vi "PlayViolins.vi"(11 "Paths to FRFs":path[](array[path])=[path "/Users/crogers/Rogers Dropbox/Chris Rogers/Violin Stuff/Violin Instruments/ME45/ME45 01/TRF/ME45 01 H_001.trf", path "/Users/crogers/Rogers Dropbox/Chris Rogers/Violin Stuff/Violin Instruments/ME45/ME45 02/TRF/ME45 02 H_001.trf", path "/Users/crogers/Rogers Dropbox/Chris Rogers/Violin Stuff/Violin Instruments/ME45/ME45 03/TRF/ME45 03 H_001.trf"]) -> ()   [LabVIEW 2024]
uses:
  <vilib>/Analysis/2dsp.llb/Inverse Complex FFT.vi
  <vilib>/Analysis/2dsp.llb/1D Convolution (DBL).vi
  <vilib>/Analysis/NI_AALPro.lvlib
  <vilib>/Analysis/NI_AALBase.lvlib
panel:
  out "Convolutions 2":waveform(dbl)[](graph)=[{"t0"=timestamp(0 s since 1904-01-01), "dt"=2.0833333333333333e-05, "Y"=array[312010 elements]}, {"t0"=timestamp(0 s since 1904-01-01), "dt"=2.0833333333333333e-05, "Y"=array[312010 elements]}, {"t0"=timestamp(0 s since 1904-01-01), "dt"=2.0833333333333333e-05, "Y"=array[312010 elements]}]
  in  "index 2":i32=48000
  in  "index":i32
  in  "Stop Button":bool
  in  "Play convolution":bool
  out "FRFs":cluster{"t0":dbl, "dt":dbl, "Y":dbl[]}[](graph)=[{"t0"=0.0, "dt"=1.0, "Y"=array[24001 elements]}, {"t0"=0.0, "dt"=1.0, "Y"=array[24001 elements]}, {"t0"=0.0, "dt"=1.0, "Y"=array[24001 elements]}]
  out "Real":T1(graph)
  out "Imaginary":T1(graph)
  in  "Play signal":bool
  in  "Path to signal":path=path "/Users/crogers/Desktop/Joseph_Convolution/1 Tchaikovsky short.wav"
  in  "musical piece":waveform(dbl)[](graph)=[{"t0"=timestamp(0 s since 1904-01-01), "dt"=2.0833333333333333e-05, "Y"=array[288010 elements]}, {"t0"=timestamp(0 s since 1904-01-01), "dt"=2.0833333333333333e-05, "Y"=array[288010 elements]}]
  out "Convolutions":waveform(dbl)[](graph)=[{"t0"=timestamp(0 s since 1904-01-01), "dt"=2.0833333333333333e-05, "Y"=array[312010 elements]}, {"t0"=timestamp(0 s since 1904-01-01), "dt"=2.0833333333333333e-05, "Y"=array[312010 elements]}, {"t0"=timestamp(0 s since 1904-01-01), "dt"=2.0833333333333333e-05, "Y"=array[312010 elements]}]
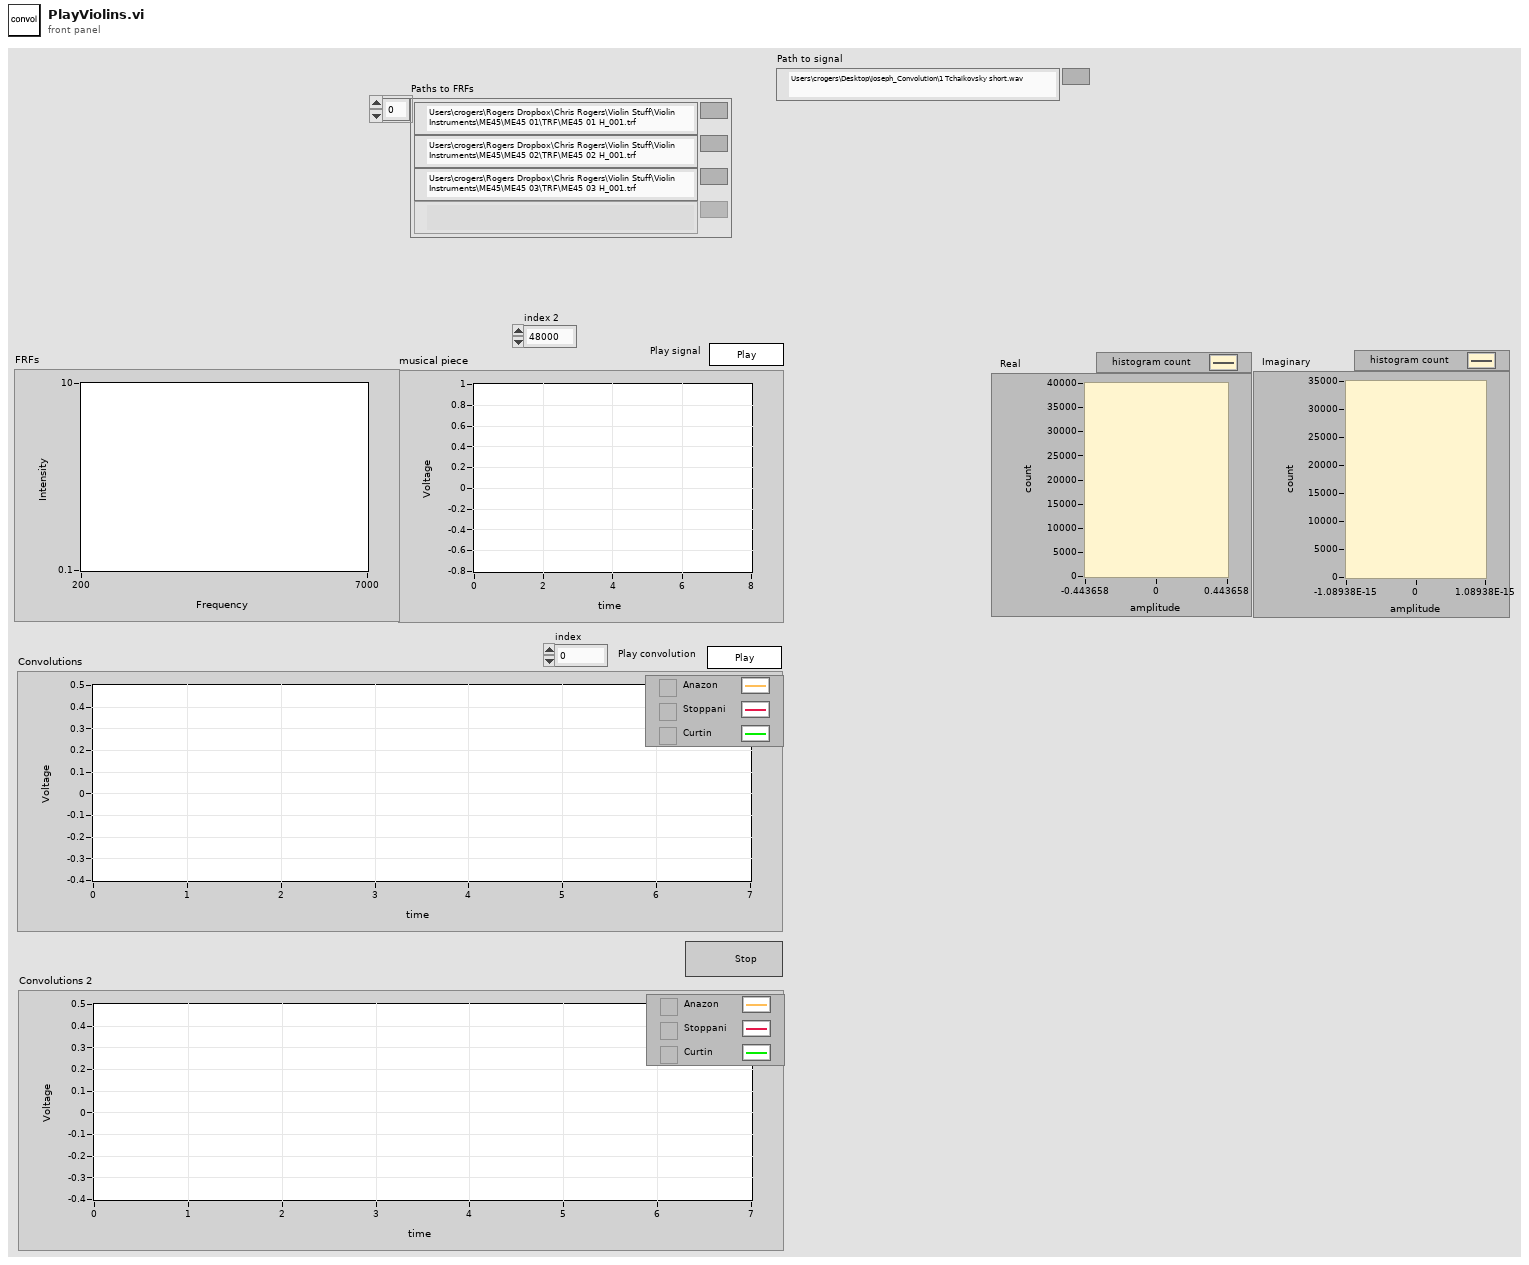
[diagram p1: front panel]
types:
  T1 = cluster{"X Values":dbl[], "Histogram: h(x)":i32[]}[]
  T2 = cluster{"X Values":dbl[], "Histogram: h(x)":i32[]}
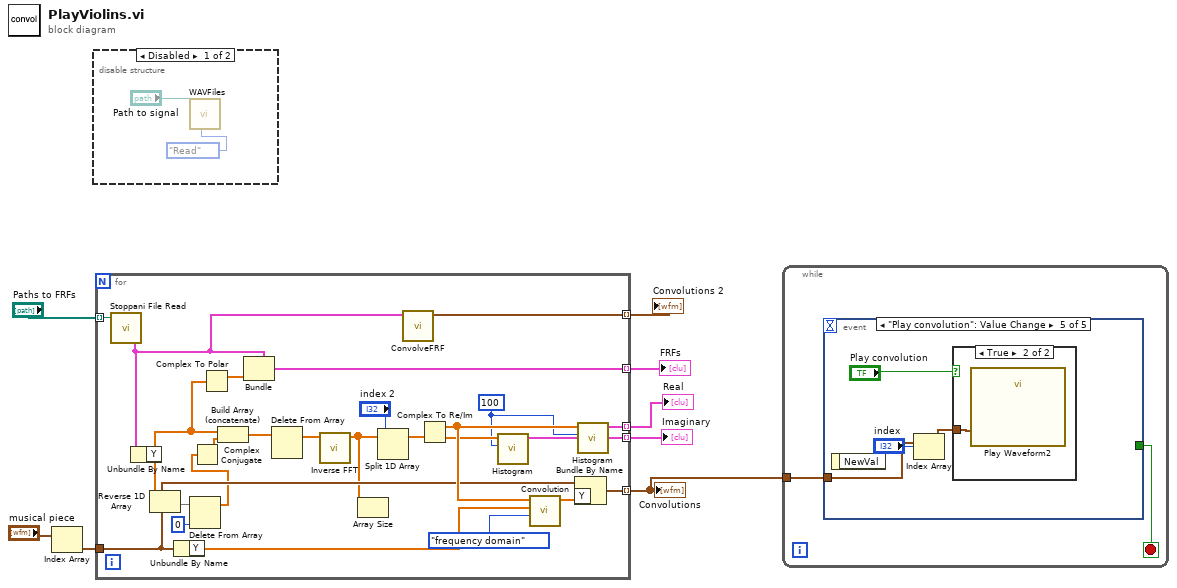
[diagram p0: block diagram]
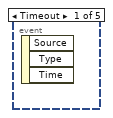
[diagram p2: hidden frame]
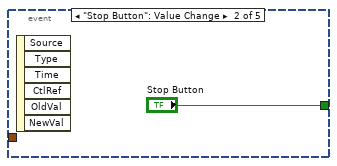
[diagram p3: hidden frame]
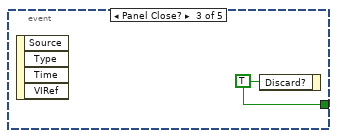
[diagram p4: hidden frame]
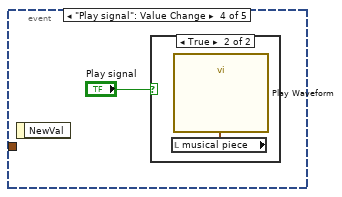
[diagram p5: hidden frame]
diagram:
  n1 = Index Array(array="musical piece") -> (element=w3:waveform(dbl))  [unwired: 1 in]
  n2 = disable-structure shown="Disabled" {
    frame Disabled {
      n3 = call "WAVFiles.vi"("Task"=enum16{"Read", "Write", "wfm"}."Read", "WAV File"="Path to signal") -> ()  [unwired: 6 in, 4 out]
    }
    frame Enabled {
    }
  }
  n4 = for {
    tunnel: [w34] -> w8 mode=indexing
    tunnel: "Paths to FRFs" -> [w33] mode=indexing
    tunnel: [w29] -> w6 mode=indexing
    tunnel: [w28] -> w5 mode=indexing
    tunnel: w3 -> [w18]
    tunnel: [w24] -> w2 mode=indexing
    tunnel: [w11] -> w1 mode=indexing
    w21 = 100 ("intervals")
    n5 = call "Stoppani File Read.vi"("String in"=w33) -> ("Complex FRF"=w12:cluster{"t0":dbl, "dt":dbl, "Y":cdb[]})  [unwired: 2 in, 3 out]
    n6 = Unbundle By Name(w12) -> ("Y"=w20:cdb[])
    n7 = Reverse 1D Array(array=w20) -> (reversed array=w31:cdb[])
    n8 = Unbundle By Name(w18) -> ("Y"=w26:dbl[])
    n9 = Delete From Array(array=w31, index=0) -> (array with subset deleted=w16:cdb[])  [unwired: 1 in, 1 out]
    n10 = Complex Conjugate(1:w16) -> (0:w15:cdb[])
    n11 = Complex To Polar(r * e^(i*theta)=w20) -> (r=w35:dbl[])  [unwired: 1 out]
    n12 = Build Array (concatenate)(w20, w15) -> (w19:cdb[])
    n13 = Bundle(cluster=w12, "Y"=w35) -> (w34:cluster{"t0":dbl, "dt":dbl, "Y":cdb[]})  [unwired: 2 in]
    n14 = Delete From Array(array=w19) -> (array with subset deleted=w30:cdb[])  [unwired: 2 in, 1 out]
    n15 = call-poly <vilib>:"Inverse FFT.vi"("FFT {X}"=w30) -> ("X"=w14:cdb[])  [unwired: 9 in, 1 out]
    n16 = Array Size(array=w14) -> ()  [unwired: 1 out]
    n17 = Split 1D Array(array=w14, index="index 2") -> (first subarray=w17:cdb[])  [unwired: 1 out]
    n18 = call "ConvolveFRF.vi"("Complex FRF"=w12) -> ("Convolution"=w11:waveform(dbl))  [unwired: 8 in, 2 out]
    n19 = Complex To Re/Im(x + iy=w17) -> (x=w23:dbl[], y=w22:dbl[])
    n20 = call <vilib>:"Histogram.vi"("intervals"=w21, "X"=w22) -> ("Histogram Graph"=w28:T2)  [unwired: 6 in, 3 out]
    n21 = call-poly <vilib>:"Convolution.vi"("algorithm"=enum32{"direct", "frequency domain"}."frequency domain", "Y"=w26, "X"=w23) -> ("X * Y"=w25:dbl[])  [unwired: 7 in, 1 out]
    n22 = Bundle By Name(cluster=w18, "Y"=w25) -> (w24:waveform(dbl))
    n23 = call <vilib>:"Histogram.vi"("intervals"=w21, "X"=w23) -> ("Histogram Graph"=w29:T2)  [unwired: 6 in, 3 out]
  }
  "FRFs" <- w8
  "Real" <- w6
  "Imaginary" <- w5
  "Convolutions" <- w2
  "Convolutions 2" <- w1
  n24 = while {
    tunnel: w2 -> [w37]
    stop <- w36 stop-if-true
    n25 = event shown="[4] \"Play convolution\": Value Change" {
      selector: _ -> [_ _ _ _ _]
      dyn-events: _ -> [_ _ _ _ _]
      timeout: _ -> [_ _ _ _ _]
      tunnel: w37 -> [_ _ _ _ w43]
      tunnel: [_ "Stop Button" w39 _ _] -> w36
      event Timeout {
        n26 = event-data() -> ()  [unwired: 1 in, 3 out]
      }
      event "Stop Button": Value Change {
        n27 = event-data() -> ()  [unwired: 1 in, 6 out]
      }
      event Panel Close? {
        w39 = TRUE ("Discard?")
        n28 = event-data() -> ()  [unwired: 1 in, 4 out]
        n29 = event-data("Discard?"=w39) -> ()  [unwired: 1 in, 1 out]
      }
      event "Play signal": Value Change {
        n30 = event-data() -> ()  [unwired: 1 in, 1 out]
        n31 = case shown="True" "Play signal" {
          frame False {
          }
          frame True {
            n32 = local read "musical piece"() -> (w41:waveform(dbl)[])
            n33 = call "Play Waveform"("Data"=w41) -> ()  [unwired: 18 in, 1 out]
          }
        }
      }
      event "Play convolution": Value Change {
        n34 = event-data() -> ()  [unwired: 1 in, 1 out]
        n35 = Index Array(array=w43, index="index") -> (element=w44:waveform(dbl))
        n36 = case shown="True" "Play convolution" {
          tunnel: w44 -> [_ w46]
          frame False {
          }
          frame True {
            n37 = call "Play Waveform2"("Data"=w46) -> ()  [unwired: 18 in, 1 out]
          }
        }
      }
    }
  }
